vi "Martins HOT interface subtract and threshold.vi"() -> ()   [LabVIEW 2012] (continued)
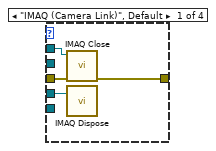
[diagram p2: hidden frame]
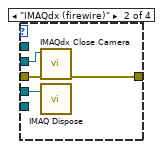
[diagram p3: hidden frame]
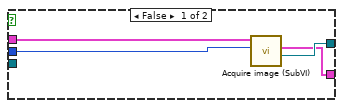
[diagram p6: hidden frame]
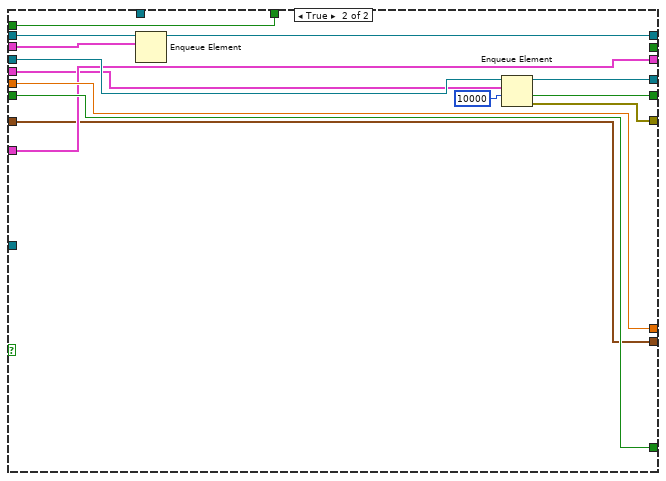
[diagram p18: hidden frame]
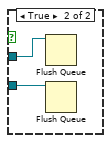
[diagram p19: hidden frame]
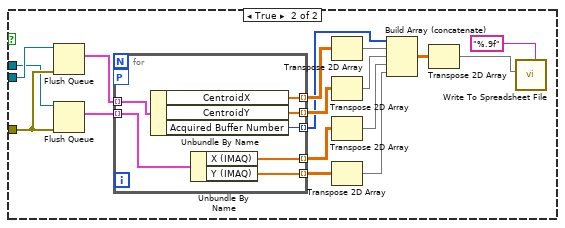
[diagram p20: hidden frame]
                  frame True {
                    n131 = local read "Coordinate mapping \n(IMAQ to SLM)"() -> (w402:T3)
                    n132 = call "Edit trap cluster.vi"("Coordinate mapping \n(IMAQ to SLM)"=w402, "trap cluster in"=w411) -> ("SubVI closed"=w406:bool, "Trap cluster out"=w405:T5)
                    n133 = Not(x=w406) -> (.not. x?=w401:bool)
                    n134 = call "Trap cluster 2 ROI.vi"("Trap cluster"=w405, "ROI in"=w403) -> ("ROI out"=w404:T2)  [unwired: 1 in]
                    n135 = property on="Monitor image" class="ImageControl"("ROI"=w404) -> ()  [unwired: 2 in, 2 out]
                    n136 = local write "Edit trap cluster"(w401) -> ()
                    n137 = Unbundle By Name(w405) -> ("Z"=w410:sgl[], "I"=w409:sgl[], "Group"=w407:bool[])
                  }
                }
                n138 = Unbundle By Name(w382) -> ("Trap number"=w381:i32[])
                n139 = case "Update display if\nnumber of traps \nhas changed" shown="True" w380 {
                  tunnel: w385 -> [_ w415]
                  tunnel: w383 -> [_ w414]
                  tunnel: w381 -> [_ w413]
                  tunnel: w378 -> [_ w412]
                  frame False {
                  }
                  frame True {
                    n140 = property on="I" class="Arr (strict)"("Value"=w414) -> ()  [unwired: 2 in, 2 out]
                    n141 = property on="Z" class="Arr (strict)"("Value"=w415) -> ()  [unwired: 2 in, 2 out]
                    n142 = property on="G" class="Arr (strict)"("Value"=w412) -> ()  [unwired: 2 in, 2 out]
                    "#" <- w413
                  }
                }
              }
              frame True {
                n143 = call "Move group.vi"("New handle position in"=w422, "Trap cluster in"=w424, "Previous handle position in"=w423, "Amplitudes"=w417, "Group"=w416, "Switch X/Y"=w418, "Move handle"=w419, "Z"=w420) -> ("Trap cluster out"=w421:T5)
              }
            }
            n144 = case shown="True" w359 {
              tunnel: w364 -> [_ w376]
              tunnel: w362 -> [w373 w375]
              tunnel: [w373 w374] -> w361
              frame False {
              }
              frame True {
                n145 = property on="Monitor image" class="ImageControl"(error in=w375, "ROI"=w376) -> (error out=w374:errorcluster)  [unwired: 1 in, 1 out]
              }
            }
          }
        }
        n146 = Wait (ms)(milliseconds to wait=u32 50) -> ()  [unwired: 1 out]
        n147 = Unbundle By Name("Path controls") -> ("Add current \npositions to path"=w341:bool, "Synchronize traps"=w350:bool, "Step length"=w353:dbl, "follow path"=w344:bool, "Arrive \nsimultaneously"=w352:bool)
        n148 = Or(x=w341, y=w350) -> (x .or. y?=w351:bool)
        n149 = Or(x=w350, y=w344) -> (x .or. y?=w348:bool)
        n150 = Or(x=w351, y=w344) -> (x .or. y?=w349:bool)
        n151 = case shown="True" "Create path" {
          tunnel: w356 -> [_ w437]
          tunnel: w346 -> [w425 w431]
          tunnel: w353 -> [_ w446]
          tunnel: w343 -> [_ w441]
          tunnel: w352 -> [_ w445]
          tunnel: w349 -> [_ w444]
          tunnel: w348 -> [_ w443]
          tunnel: w344 -> [_ w442]
          tunnel: w345 -> [w428 w438]
          tunnel: w340 -> [_ w436]
          tunnel: w339 -> [_ w435]
          tunnel: w337 -> [w427 w434]
          tunnel: [w427 w433] -> w336
          tunnel: "Updating trap cluster" -> [w426 _]
          tunnel: [w425 w432] -> w334
          frame False {
            n152 = case shown="True" w426 {
              tunnel: w425 -> [_ w430]
              tunnel: w428 -> [_ w429]
              frame False {
              }
              frame True {
                n153 = Lossy Enqueue Element(queue=w429, element=w430) -> ()  [unwired: 1 in, 4 out]
              }
            }
          }
          frame True {
            n154 = Lossy Enqueue Element "Enqueue\noverlay pos"(queue=w436, element=w431) -> ()  [unwired: 1 in, 4 out]
            n155 = case "Add wpt" shown="True" w444 {
              tunnel: w431 -> [_ w523]
              tunnel: w437 -> [w520 w524]
              tunnel: [w520 w521] -> w447
              tunnel: [_ w522] -> w439
              frame False {
              }
              frame True {
                n156 = Enqueue Element "Enqueue path\n waypts"(queue=w524, element=w523) -> (queue out=w521:refnum<queue>, error out=w522:errorcluster)  [unwired: 2 in, 1 out]
              }
            }
            n157 = case "Compute path" shown="True" w443 {
              tunnel: w447 -> [_ w531]
              tunnel: w441 -> [_ w530]
              tunnel: w446 -> [_ w529]
              tunnel: w445 -> [_ w528]
              tunnel: [w525 w526] -> w440
              tunnel: w439 -> [w525 w527]
              frame False {
              }
              frame True {
                n158 = call "compute path cluster.vi"("path queue"=w530, "Arrive simultaeously"=w528, "error in (no error)"=w527, "Step length\n(IMAQ pixels)"=w529, "waypoint queue"=w531) -> ("error out"=w526:errorcluster)  [unwired: 2 in]
              }
            }
            n159 = case "Follow path" shown="True" w442 {
              tunnel: w441 -> [_ w476]
              tunnel: w440 -> [_ w477]
              tunnel: w438 -> [_ w479]
              tunnel: w437 -> [_ w478]
              tunnel: w435 -> [_ w475]
              tunnel: w434 -> [w449 w456]
              tunnel: [w449 w455] -> w433
              tunnel: [w448 w450] -> w432
              tunnel: w431 -> [w448 _]
              frame False {
              }
              frame True {
                w470 = TRUE ("Visible")
                n160 = local write "Display path"(FALSE ("Display path")) -> ()
                n161 = Flush Queue "Flush Waypts"(queue=w478, error in (no error)=w477) -> (error out=w469:errorcluster)  [unwired: 2 out]
                n162 = Get Queue Status(queue=w476, error in (no error)=w469) -> (queue out=w473:refnum<queue>, error out=w468:errorcluster, # elements in queue=w472:i32)  [unwired: 1 in, 5 out]
                n163 = property on="Pause" class="Bool (strict)"(error in=w468, "Visible"=w470) -> (error out=w467:errorcluster)  [unwired: 1 in, 1 out]
                n164 = property on="cancel path" class="Bool"(error in=w467, "Visible"=w470) -> (error out=w466:errorcluster)  [unwired: 1 in, 1 out]
                n165 = for {
                  N: w472 -> [_]
                  tunnel: w466 -> [w498]
                  tunnel: w479 -> [w500]
                  tunnel: w473 -> [w496]
                  tunnel: [w496] -> w471
                  tunnel: [FALSE ("Group traps")] -> w451
                  shift-right: [w487] -> w450
                  shift-left: _ -> [w489]
                  tunnel: [w486] -> w465
                  tunnel: [w483] -> w463 mode=indexing
                  tunnel: [w484] -> w459
                  tunnel: [TRUE ("Display path")] -> w457
                  i -> [w484]
                  stop <- w493 stop-if-true
                  n166 = Dequeue Element(queue=w496, timeout in ms (-1)=0, error in (no error)=w498) -> (element=w488:T5, timed out?=w492:bool, error out=w499:errorcluster)  [unwired: 1 out]
                  n167 = while {
                    tunnel: [w517] -> w490
                    tunnel: ["cancel path"] -> w485
                    stop <- w519 stop-if-true
                    n168 = local read "Stop program"() -> (w517:bool)
                    n169 = Wait (ms)(milliseconds to wait="Step time \n(ms)") -> ()  [unwired: 1 out]
                    n170 = Or(x=w517, y="cancel path") -> (x .or. y?=w515:bool)
                    n171 = Implies(1:w515, 2:"Pause") -> (0:w519:bool)
                  }
                  n172 = case shown="True" "Skip step if \ntimed out" {
                    tunnel: w500 -> [w506 w511]
                    tunnel: w499 -> [w505 w509]
                    tunnel: [FALSE ("overflow?") w507] -> w491
                    tunnel: w488 -> [w504 w510]
                    tunnel: [w503 w508] -> w486
                    tunnel: 500 ("timeout in ms (-1)") -> [w502 _]
                    frame False {
                      n173 = Enqueue Element "Enqueue trap pos"(queue=w506, element=w504, timeout in ms (-1)=w502, error in (no error)=w505) -> (error out=w503:errorcluster)  [unwired: 2 out]
                    }
                    frame True {
                      n174 = Lossy Enqueue Element(queue=w511, element=w510, error in (no error)=w509) -> (overflow?=w507:bool, error out=w508:errorcluster)  [unwired: 2 out]
                    }
                  }
                  "Step skipped" <- w491
                  n175 = case shown="False" w490 {
                    tunnel: w489 -> [_ w513]
                    tunnel: w488 -> [w512 _]
                    tunnel: [w512 w513] -> w487
                    frame False {
                    }
                    frame True {
                    }
                  }
                  n176 = Or(x=w485, y=w490) -> (x .or. y?=w495:bool)
                  n177 = Or(x=w495, y=w492) -> (x .or. y?=w493:bool)
                  n178 = Tick Count (ms)() -> (millisecond timer value=w483:u32)
                }
                n179 = local read "Transpose SLM"() -> (w453:bool)
                n180 = call "Trap cluster 2 ROI.vi"("Switch X/Y"=w453, "Trap cluster"=w450, "ROI in"=w475) -> ("ROI out"=w474:T2)
                n181 = local write "Step skipped"(w451) -> ()
                n182 = local write "Create path"(w451) -> ()
                n183 = local write "Display path"(w457) -> ()
                n184 = local write "Group \nTraps"(w451) -> ()
                n185 = property on="Pause" class="Bool (strict)"(error in=w465, "Visible"=w451, "Value"=w451) -> (error out=w464:errorcluster)  [unwired: 1 in, 1 out]
                n186 = property on="cancel path" class="Bool"(error in=w464, "Visible"=w451) -> ()  [unwired: 1 in, 2 out]
                n187 = property on="follow path" class="Bool (strict)"("Value"=w451) -> ()  [unwired: 2 in, 2 out]
                n188 = property on="Monitor image" class="ImageControl"(error in=w456, "ROI"=w474) -> (error out=w455:errorcluster)  [unwired: 1 in, 1 out]
                n189 = Array Max & Min(array=w463) -> (max value=w462:u32, min value=w461:u32)  [unwired: 2 out]
                n190 = Subtract(x=w462, y=w461) -> (x-y=w460:u32)
                n191 = Increment(x=w459) -> (x+1=w454:i32)
                n192 = Divide(x=w460, y=w454) -> (x/y=→"Average step time (ms)":dbl)
                n193 = Flush Queue "Flush Path"(queue=w471) -> ()  [unwired: 1 in, 3 out]
              }
            }
          }
        }
        n194 = First Call?() -> (First Call?: T/F=w331:bool)
        n195 = Or(x="Apply Corrections", y=w331) -> (x .or. y?=w332:bool)
        n196 = case shown="True" w332 {
          frame False {
          }
          frame True {
            n197 = call "Apply Corrections.vi"() -> ()  [unwired: 1 in]
          }
        }
      }
      frame True {
        n198 = property on="Cancel calibration" class="Bool"("Visible"=w534) -> ()  [unwired: 2 in, 2 out]
        n199 = flat-sequence {
          tunnel: [w559] -> w546
          tunnel: [w561] -> w545
          tunnel: w541 -> [w559]
          tunnel: [w551] -> w540
          tunnel: [w548] -> w539
          tunnel: w538 -> [w553]
          tunnel: [w552] -> w536
          tunnel: [w624] -> w544
          tunnel: w546 -> [w624]
          tunnel: w545 -> [w582]
          tunnel: [w620] -> w543
          tunnel: w542 -> [w623]
          tunnel: w540 -> [w622]
          tunnel: w539 -> [w619]
          tunnel: [w618] -> w537
          tunnel: w536 -> [w618]
          tunnel: [w580] -> w532
          tunnel: w544 -> [w689]
          tunnel: w537 -> [w687]
          tunnel: [w686] -> w535
          frame #0 {
            w562 = u32 8 items=["Zoom Tool"=8, "Selection Tool"=0, "Pan Tool"=9, "Point Tool"=1, "Line Tool"=2, "Rectangle Tool"=3, "Rotated Rectangle Tool"=12, "Polyline Tool"=10, "Polygon Tool"=5, "Freehand Tool"=11, "Closed Freehand Tool"=6, "Ellipse Tool"=4, "Annulus Tool"=7] ("Current ROI Tool")
            n200 = local read "Using monitoring camera\nfor measurements"() -> (w547:bool)
            n201 = local read "Coordinate mapping \n(IMAQ to SLM)"() -> (w548:T3)
            n202 = Bundle By Name(cluster=w548, "sX"=0.0, "sY"=0.0, "cX"=1.0 ("sX"), "cY"=1.0) -> (w551:T3)
            n203 = case shown="False" w547 {
              frame False {
                n204 = call <vilib>:"Application Directory.vi"() -> ("Application Directory"=w565:path)
                n205 = Build Path(base path=w565, name or relative path="Sub VIs\\Display Image.vi") -> (appended path=w568:path)
                n206 = Open VI Reference(vi path=w568) -> (vi reference=w567:refnum<vi>)  [unwired: 5 in, 1 out]
                n207 = property class="VI"(reference=w567, "Front Panel.Open"=TRUE ("Front Panel Window:Open")) -> ()  [unwired: 1 in, 2 out]
              }
              frame True {
              }
            }
            n208 = local write "Coordinate mapping \n(IMAQ to SLM)"(w551) -> ()
            n209 = property on="ok" class="Bool"("Visible"=TRUE ("ROI Tool Buttons Visibile:Zoom Tool Button Visible")) -> ()  [unwired: 2 in, 2 out]
            n210 = property on="Monitor image" class="ImageControl"("Current ROI Tool"=w562) -> ()  [unwired: 2 in, 2 out]
            n211 = call <vilib>:"Three Button Dialog.vi"("Center Button Text (\"No\")"="Manual" ("T button name (\"OK\")"), "Left Button Text (\"Yes\")"="Auto" ("F button name (\"Cancel\")"), "message"="Mark the center of the \ndisplayed spot using the \nzoom and the point tool, \nthen click the OK button. \n(Will be repeated three times)") -> ("Which Button?"=w561:T13)  [unwired: 8 in]
            n212 = property on="Monitor image" class="ImageControl"(error in=w553, "ROI"=T2 {"Global Rectangle"=[100, 100, 394, 354], "Contours"=[{"Contour Type"=0, "ROI Type"=1, "Points"=[100, 100]}]} ("ROI 2")) -> (error out=w552:errorcluster)  [unwired: 1 in, 1 out]
          }
          frame #1 {
            w576 = sgl 0.0 ("sX")
            w577 = sgl 1.0 ("cX")
            n213 = local read "Coordinate mapping \n(Monitor to Measurement)"() -> (w575:T3)
            n214 = for {
              tunnel: [w645] -> w613 mode=indexing
              tunnel: [w644] -> w612 mode=indexing
              tunnel: T5[] [{"X (IMAQ)"=[-85.0], "Y (IMAQ)"=[-85.0], "Z"=[0.0], "I"=[100.0], "Trap number"=[0], "ROI number"=[0], "Number of traps"=1, "Group"=[]}, {"X (IMAQ)"=[85.0], "Y (IMAQ)"=[-85.0], "Z"=[0.0], "I"=[100.0], "Trap number"=[0], "ROI number"=[0], "Number of traps"=1, "Group"=[]}, {"X (IMAQ)"=[-85.0], "Y (IMAQ)"=[85.0], "Z"=[0.0], "I"=[100.0], "Trap number"=[0], "ROI number"=[0], "Number of traps"=0, "Group"=[]}] -> [w643] mode=indexing
              tunnel: [w640] -> w600 mode=indexing
              tunnel: [w638] -> w599 mode=indexing
              tunnel: w623 -> [w642]
              tunnel: [w637] -> w588 mode=indexing
              tunnel: [w636] -> w587 mode=indexing
              tunnel: w582 -> [w635]
              tunnel: [w633] -> w581
              stop <- w634 stop-if-true
              n215 = Enqueue Element "Enqueue trap pos"(queue=w642, element=w643) -> ()  [unwired: 2 in, 3 out]
              n216 = case shown="\"Left Button\", Default" w635 {
                tunnel: [w650 w667 _ _] -> w645
                tunnel: [w649 w666 _ _] -> w644
                tunnel: [w646 w664 w677 w678] -> w634
                tunnel: [w648 w661 _ _] -> w637
                tunnel: [w647 w660 _ _] -> w636
                tunnel: [w646 w659 w677 w678] -> w633
                frame "Left Button", Default {
                  n217 = flat-sequence {
                    tunnel: [w658] -> w650
                    tunnel: [w657] -> w649
                    tunnel: [w656] -> w648
                    tunnel: [w655] -> w647
                    tunnel: [FALSE] -> w646
                    frame #0 {
                      n218 = Wait (ms)(milliseconds to wait=u32 300) -> ()  [unwired: 1 out]
                    }
                    frame #1 {
                      n219 = local read "Monitoring image"() -> (w654:T1)
                      n220 = local read "Measurement image"() -> (w653:T1)
                      n221 = call "Find spot in image.vi"("Image"=w654) -> ("Y Centroid"=w657:dbl, "X Centroid"=w658:dbl)  [unwired: 7 in]
                      n222 = call "Find spot in image.vi"("Image"=w653) -> ("Y Centroid"=w655:dbl, "X Centroid"=w656:dbl)  [unwired: 7 in]
                    }
                  }
                }
                frame "Center Button" {
                  n223 = while {
                    tunnel: [w675] -> w665
                    tunnel: [w672] -> w664
                    tunnel: [w670] -> w663
                    tunnel: [w669] -> w659
                    stop <- w673 stop-if-true
                    n224 = local read "Stop program"() -> (w669:bool)
                    n225 = global read "Global variables.vi" "Measurement ROI"() -> (w670:T14)
                    n226 = Wait (ms)(milliseconds to wait=u32 50) -> ()  [unwired: 1 out]
                    n227 = Or(x=w669, y="Cancel calibration") -> (x .or. y?=w672:bool)
                    n228 = property on="Monitor image" class="ImageControl"() -> ("ROI"=w675:T2)  [unwired: 2 in, 2 out]
                    n229 = Or(x="ok", y=w672) -> (x .or. y?=w673:bool)
                  }
                  n230 = Unbundle By Name(w663) -> ("Global Rectangle"=w662:i32[])  [unwired: 1 out]
                  n231 = Unbundle By Name(w665) -> ("Global Rectangle"=w668:i32[])  [unwired: 1 out]
                  n232 = Index Array(array=w668) -> (element #1=w667:i32, element #2=w666:i32)  [unwired: 2 in]
                  n233 = Index Array(array=w662) -> (element #1=w661:i32, element #2=w660:i32)  [unwired: 2 in]
                }
                frame "Right Button" {
                  w677 = TRUE
                }
                frame "Window Close" {
                  w678 = TRUE
                }
              }
              n234 = Unbundle By Name(w643) -> ("X (IMAQ)"=w641:sgl[], "Y (IMAQ)"=w639:sgl[])
              n235 = Index Array(array=w639) -> (element=w638:sgl)  [unwired: 1 in]
              n236 = Index Array(array=w641) -> (element=w640:sgl)  [unwired: 1 in]
            }
            n237 = Index Array(array=w612) -> (element #1=w614:dbl, element #2=w615:dbl)  [unwired: 2 in]
            n238 = Index Array(array=w613) -> (element #1=w616:dbl, element #2=w617:dbl)  [unwired: 2 in]
            n239 = Subtract(x=w617, y=w616) -> (x-y=w609:dbl)
            n240 = Subtract(x=w615, y=w614) -> (x-y=w607:dbl)
            n241 = Absolute Value(x=w607) -> (abs(x)=w606:dbl)
            n242 = Absolute Value(x=w609) -> (abs(x)=w608:dbl)
            n243 = Less?(x=w608, y=w606) -> (x < y?=w571:bool)
            n244 = case shown="False" w571 {
              tunnel: w613 -> [w630 w632]
              tunnel: w612 -> [w629 w631]
              tunnel: [w629 w632] -> w610
              tunnel: [w630 w631] -> w611
              frame False {
              }
              frame True {
              }
            }
            n245 = Index Array(array=w587) -> (element #1=w592:dbl, element #2=w591:dbl)  [unwired: 2 in]
            n246 = Index Array(array=w588) -> (element #1=w590:dbl, element #2=w589:dbl)  [unwired: 2 in]
            n247 = Subtract(x=w589, y=w590) -> (x-y=w593:dbl)
            n248 = Subtract(x=w591, y=w592) -> (x-y=w595:dbl)
            n249 = Absolute Value(x=w595) -> (abs(x)=w596:dbl)
            n250 = Absolute Value(x=w593) -> (abs(x)=w594:dbl)
            n251 = Less?(x=w594, y=w596) -> (x < y?=w572:bool)
            n252 = case shown="True" w572 {
              tunnel: w588 -> [w626 w628]
              tunnel: w587 -> [w625 w627]
              tunnel: [w625 w628] -> w597
              tunnel: [w626 w627] -> w598
              frame False {
              }
              frame True {
              }
            }
            n253 = formula code="cX = (xSLM[1] - xSLM[0]) / (xMonitor[1] - xMonitor[0]); \ncY = (ySLM[2] - ySLM[0]) / (yMonitor[2] - yMonitor[0]); \n\nsX = xSLM[0] - xMonitor[0] *cX;\nsY = ySLM[0] - yMonitor[0] *cY;\n\ncXm = (xMeasure[1] - xMeasure[0]) / (xMonitor[1] - xMonitor[0]); \ncYm = (yMeasure[2] - yMeasure[0]) / (yMonitor[2] - yMonitor[0]); \n\nsXm = xMeasure[0] - xMonitor[0] *cXm;\nsYm = yMeasure[0] - yMonitor[0] *cYm;"("xMonitor"=w611, "yMonitor"=w610, "xSLM"=w600, "ySLM"=w599, "xMeasure"=w598, "yMeasure"=w597) -> ("cX"=w605:dbl, "cY"=w604:dbl, "sX"=w603:dbl, "sY"=w602:dbl, "cXm"=w586:dbl, "cYm"=w585:dbl, "sXm"=w584:dbl, "sYm"=w583:dbl)
            n254 = local read "Using monitoring camera\nfor measurements"() -> (w570:bool)
            n255 = Select(t=FALSE, s=w570, f=w572) -> (s? t:f=w573:bool)
            n256 = Bundle By Name(cluster=w622, "cX"=w605, "cY"=w604, "sX"=w603, "sY"=w602) -> (w621:T3)
            n257 = Bundle By Name(cluster=w575, "cX"=w577, "cY"=w577, "sX"=w576, "sY"=w576) -> (w574:T3)
            n258 = Bundle By Name(cluster=w575, "cX"=w586, "cY"=w585, "sX"=w584, "sY"=w583) -> (w578:T3)
            n259 = Select(t=w574, s=w570, f=w578) -> (s? t:f=w579:T3)
            n260 = case "Calibration canceled?" shown="False" w581 {
              tunnel: w621 -> [w682 _]
              tunnel: [w682 w684] -> w620
              tunnel: w619 -> [_ w684]
              tunnel: [w679 w683] -> w580
              tunnel: w579 -> [w679 w683]
              tunnel: w573 -> [w681 _]
              tunnel: w571 -> [w680 _]
              frame False {
                n261 = local write "Transpose Measurement"(w681) -> ()
                n262 = local write "Transpose SLM"(w680) -> ()
              }
              frame True {
              }
            }
          }
          frame #2 {
            w685 = FALSE ("ROI Tool Buttons Visibile:Zoom Tool Button Visible")
            w688 = u32 1 items=["Zoom Tool"=8, "Selection Tool"=0, "Pan Tool"=9, "Point Tool"=1, "Line Tool"=2, "Rectangle Tool"=3, "Rotated Rectangle Tool"=12, "Polyline Tool"=10, "Polygon Tool"=5, "Freehand Tool"=11, "Closed Freehand Tool"=6, "Ellipse Tool"=4, "Annulus Tool"=7] ("Current ROI Tool")
            n263 = property on="Monitor image" class="ImageControl"(error in=w687, "ROI"=w689) -> (error out=w686:errorcluster)  [unwired: 1 in, 1 out]
            n264 = property on="Monitor image" class="ImageControl"("Current ROI Tool"=w688, "Point Tool Button Visibile"=w685) -> ()  [unwired: 2 in, 2 out]
            n265 = property on="Cancel" class="Bool"("Visible"=w685) -> ()  [unwired: 2 in, 2 out]
            n266 = property on="ok" class="Bool"("Visible"=w685) -> ()  [unwired: 2 in, 2 out]
          }
        }
        n267 = local write "Coordinate mapping \n(IMAQ to SLM)"(w543) -> ()
        n268 = local write "Coordinate mapping \n(Monitor to Measurement)"(w532) -> ()
      }
    }
  }
  n269 = while "User input and events loop" {
    tunnel: w73 -> [w708]
    tunnel: w12 -> [w697]
    tunnel: w47 -> [w696]
    tunnel: w11 -> [w695]
    tunnel: [w694] -> w56
    tunnel: w55 -> [w693]
    tunnel: [w692] -> w54
    tunnel: w37 -> [w690]
    stop <- w700 stop-if-true
    w705 = u32 8 items=["Zoom Tool"=8, "Selection Tool"=0, "Pan Tool"=9, "Point Tool"=1, "Line Tool"=2, "Rectangle Tool"=3, "Rotated Rectangle Tool"=12, "Polyline Tool"=10, "Polygon Tool"=5, "Freehand Tool"=11, "Closed Freehand Tool"=6, "Ellipse Tool"=4, "Annulus Tool"=7] ("Current ROI Tool")
    w702 = T15 [enum."LCONTROL"] items=["0", "1", "2", "3", "4", "5", "6", "7", "8", "9", "A", "B", "C", "D", "E", "F", "G", "H", "I", "J", "K", "L", "M", "N", "O", "P", "Q", "R", "S", "T", "U", "V", "W", "X", "Y", "Z", "F1", "F2", "F3", "F4", "F5", "F6", "F7", "F8", "F9", "F10", "F11", "F12", "F13", "F14", "F15", "ADD", "BACK", "BACKSLASH", "CAPITAL", "COMMA", "DECIMAL", "DELETE", "DIVIDE", "DOWN", "END", "EQUALS", "ESCAPE", "GRAVE (`)", "HOME", "INSERT", "LBRACKET", "LCONTROL", "LEFT", "L ALT", "LSHIFT", "LWIN", "MINUS", "MULTIPLY", "NEXT", "NUMLOCK", "NUMPAD_0", "NUMPAD_1", "NUMPAD_2", "NUMPAD_3", "NUMPAD_4", "NUMPAD_5", "NUMPAD_6", "NUMPAD_7", "NUMPAD_8", "NUMPAD_9", "PAUSE", "PERIOD", "PRIOR (PG UP)", "RBRACKET", "RCONTROL", "RETURN", "RIGHT", "R ALT", "RSHIFT", "RWIN", "SCROLL", "SEMICOLON", "SLASH", "SPACE", "SUBTRACT", "TAB", "UP", "ENTER (num pad)", "' (quote)"] ("keys pressed")
    n270 = call-poly <vilib>:"Acquire Input Data.vi"("device ID"=w708, "error in (no error)"=w693) -> ("device ID"=w694:refnum<k1>, "keys pressed"=w701:T15, "error out"=w692:errorcluster)  [unwired: 15 out]
    n271 = property on="Monitor image" class="ImageControl"() -> ("Current ROI Tool"=w704:u32)  [unwired: 2 in, 2 out]
    n272 = Equal?(x=w701, y=w702) -> (x = y?=w703:bool[])
    n273 = Not Equal?(x=w704, y=w705) -> (x != y?=w706:bool)
    n274 = Or Array Elements(Boolean array=w703) -> (logical OR=w707:bool)
    n275 = case shown="True" w706 {
      tunnel: w707 -> [_ w753]
      frame False {
      }
      frame True {
        n276 = case shown="False" w753 {
          frame False {
            w754 = u32 0 items=["Zoom Tool"=8, "Selection Tool"=0, "Pan Tool"=9, "Point Tool"=1, "Line Tool"=2, "Rectangle Tool"=3, "Rotated Rectangle Tool"=12, "Polyline Tool"=10, "Polygon Tool"=5, "Freehand Tool"=11, "Closed Freehand Tool"=6, "Ellipse Tool"=4, "Annulus Tool"=7] ("Current ROI Tool")
            n277 = property on="Monitor image" class="ImageControl"("Current ROI Tool"=w754) -> ()  [unwired: 2 in, 2 out]
          }
          frame True {
            w755 = u32 1 items=["Zoom Tool"=8, "Selection Tool"=0, "Pan Tool"=9, "Point Tool"=1, "Line Tool"=2, "Rectangle Tool"=3, "Rotated Rectangle Tool"=12, "Polyline Tool"=10, "Polygon Tool"=5, "Freehand Tool"=11, "Closed Freehand Tool"=6, "Ellipse Tool"=4, "Annulus Tool"=7] ("Current ROI Tool")
            n278 = property on="Monitor image" class="ImageControl"("Current ROI Tool"=w755) -> ()  [unwired: 2 in, 2 out]
          }
        }
      }
    }
    n279 = Wait (ms)(milliseconds to wait=u32 50) -> ()  [unwired: 1 out]
    n280 = case shown="False" "View Licence" {
      frame False {
      }
      frame True {
        n281 = call "View license.vi"() -> ()  [unwired: 1 in]
      }
    }
    n282 = event shown="[0] Timeout" {
      selector: _ -> [_ _ _ _ _ _ _ _ _ _ _]
      dyn-events: _ -> [_ _ _ _ _ _ _ _ _ _ _]
      timeout: 0 -> [_ _ _ _ _ _ _ _ _ _ _]
      tunnel: w697 -> [_ _ w719 _ _ _ _ _ _ _ _]
      tunnel: w696 -> [_ _ w718 _ _ _ _ _ _ _ _]
      tunnel: w695 -> [_ _ w722 _ _ _ _ _ _ _ _]
      tunnel: w690 -> [_ _ _ _ _ _ w735 _ _ _ _]
      event Timeout {
        n283 = event-data() -> ()  [unwired: 1 in, 2 out]
      }
      event "Display hologram\nand computed \nimage plane": Value Change {
        n284 = event-data() -> ("NewVal"=w710:bool)  [unwired: 1 in, 4 out]
        n285 = property on="Current trap pos" class="Clust (strict)"("Visible"=w710) -> ()  [unwired: 2 in, 2 out]
        n286 = property on="Displayed Hologram" class="IntGraph (strict)"("Visible"=w710) -> ()  [unwired: 2 in, 2 out]
        n287 = property on="Calculated image plane" class="IntGraph (strict)"("Visible"=w710) -> ()  [unwired: 2 in, 2 out]
        n288 = property on="Property Node" class="VI"() -> ("Front Panel.WinBounds"=w717:T16)  [unwired: 2 in, 2 out]
        n289 = Unbundle By Name(w717) -> ("Right"=w716:i16, "Left"=w715:i16)
        n290 = Subtract(x=w716, y=w715) -> (x-y=w714:i16)
        n291 = Select(t=i16 500 ("x-y"), s=w710, f=i16 196 ("x-y")) -> (s? t:f=w709:i16)
        n292 = Subtract(x=w714, y=w709) -> (x-y=w713:i16)
        n293 = property on="Splitter" class="Splitter"("Position"=w713) -> ()  [unwired: 2 in, 2 out]
      }
      event "Create path": Value Change {
        n294 = event-data() -> ()  [unwired: 1 in, 5 out]
        n295 = property on="follow path" class="Bool (strict)"("Value"=FALSE) -> ()  [unwired: 2 in, 2 out]
        n296 = Flush Queue "Flush path \nwaypt queue"(queue=w718) -> ()  [unwired: 1 in, 3 out]
        n297 = Preview Queue Element(queue=w719) -> (element=w720:T5, error out=w723:errorcluster)  [unwired: 2 in, 2 out]
        n298 = Flush Queue "Flush path queue"(queue=w722) -> (queue out=w721:refnum<queue>)  [unwired: 1 in, 2 out]
        n299 = Enqueue Element "Enqueue current \ntrap pos in path"(queue=w721, element=w720) -> ()  [unwired: 2 in, 3 out]
        n300 = Enqueue Element "Enqueue current \ntrap pos in path \nwaypts"(queue=w718, element=w720, error in (no error)=w723) -> ()  [unwired: 1 in, 3 out]
      }
      event "cancel path": Value Change {
        n301 = event-data() -> ()  [unwired: 1 in, 5 out]
        n302 = local write "Create path"(FALSE ("Visible")) -> ()
      }
      event "Monitor image", "Group \nTraps", "Z", "I", "Coordinate mapping \n(IMAQ to SLM)": Mouse Down {
        w726 = FALSE ("Edit trap cluster")
        n303 = event-data() -> ()  [unwired: 1 in, 7 out]
        n304 = local write "Updating trap cluster"(TRUE ("Update trap positions")) -> ()
        n305 = local write "Edit trap cluster"(w726) -> ()
        n306 = call <vilib>:"Application Directory.vi"() -> ("Application Directory"=w727:path)
        n307 = Build Path(base path=w727, name or relative path="Sub VIs\\Edit trap cluster.vi") -> (appended path=w730:path)
        n308 = Open VI Reference(vi path=w730) -> (vi reference=w729:refnum<vi>)  [unwired: 5 in, 1 out]
        n309 = property class="VI"(reference=w729, "Front Panel.Open"=w726) -> ()  [unwired: 1 in, 2 out]
      }
      event "Group \nTraps", "Z", "I", "Monitor image", "Coordinate mapping \n(IMAQ to SLM)": Mouse Up {
        n310 = event-data() -> ()  [unwired: 1 in, 7 out]
        n311 = flat-sequence {
          frame #0 {
            n312 = Wait (ms)(milliseconds to wait=u32 100) -> ()  [unwired: 1 out]
          }
          frame #1 {
            n313 = local write "Updating trap cluster"(FALSE ("Update trap positions")) -> ()
          }
        }
      }
      event "Record": Value Change {
        n314 = event-data() -> ()  [unwired: 1 in, 5 out]
        n315 = Unbundle By Name(w735) -> ("Image buffers"=w734:T1[])
        n316 = for {
          tunnel: w734 -> [w736] mode=indexing
          n317 = call "IMAQ Clear Overlay"("Image"=w736) -> ()  [unwired: 9 in, 2 out]
        }
      }
      event "Display data": Value Change {
        n318 = event-data() -> ("NewVal"=w738:bool)  [unwired: 1 in, 4 out]
        n319 = call <vilib>:"Application Directory.vi"() -> ("Application Directory"=w737:path)
        n320 = Build Path(base path=w737, name or relative path="Sub VIs\\Display Cetroids (SubVI).vi") -> (appended path=w741:path)
        n321 = Open VI Reference(vi path=w741) -> (vi reference=w740:refnum<vi>)  [unwired: 5 in, 1 out]
        n322 = property class="VI"(reference=w740, "Front Panel.Open"=w738) -> ()  [unwired: 1 in, 2 out]
      }
      event "Display ROIs": Value Change {
        n323 = event-data() -> ("NewVal"=w742:bool)  [unwired: 1 in, 4 out]
        n324 = call <vilib>:"Application Directory.vi"() -> ("Application Directory"=w743:path)
        n325 = Build Path(base path=w743, name or relative path="Sub VIs\\Display ROIs.vi") -> (appended path=w746:path)
        n326 = Open VI Reference(vi path=w746) -> (vi reference=w745:refnum<vi>)  [unwired: 5 in, 1 out]
        n327 = property class="VI"(reference=w745, "Front Panel.Open"=w742) -> ()  [unwired: 1 in, 2 out]
      }
      event "Display ROIs": Value Change {
        n328 = event-data() -> ("NewVal"=w747:bool)  [unwired: 1 in, 4 out]
        n329 = call <vilib>:"Application Directory.vi"() -> ("Application Directory"=w748:path)
        n330 = Build Path(base path=w748, name or relative path="Sub VIs\\Display Image.vi") -> (appended path=w751:path)
        n331 = Open VI Reference(vi path=w751) -> (vi reference=w750:refnum<vi>)  [unwired: 5 in, 1 out]
        n332 = property class="VI"(reference=w750, "Front Panel.Open"=w747) -> ()  [unwired: 1 in, 2 out]
      }
      event "Edit trap cluster": Value Change {
        n333 = event-data() -> ("NewVal"=w752:bool)  [unwired: 1 in, 4 out]
        n334 = local write "Updating trap cluster"(w752) -> ()
      }
    }
    n335 = local read "Stop program"() -> (w700:bool)
  }
  n336 = Unbundle By Name(w26) -> ("Camera type"=w16:T8)
  n337 = local read "Using monitoring camera\nfor measurements"() -> (w15:bool)
  n338 = call "IMAQ Create"("Image Name"="Monitoring copy", "Image Type"=w6) -> ("New Image"=w13:T1)  [unwired: 3 in, 1 out]
  n339 = while {
    tunnel: w26 -> [w773]
    tunnel: [w771] -> w17
    tunnel: w16 -> [w772]
    tunnel: w15 -> [w769]
    tunnel: w13 -> [w768]
    tunnel: w12 -> [w767]
    tunnel: w11 -> [w761]
    tunnel: w10 -> [w756]
    stop <- w774 stop-if-true
    n340 = Preview Queue Element(queue=w767, timeout in ms (-1)=10) -> (element=w766:T5)  [unwired: 1 in, 3 out]
    n341 = case shown="True" w769 {
      tunnel: w773 -> [w779 w782]
      tunnel: w772 -> [w778 _]
      tunnel: [w777 w783] -> w765
      tunnel: [w776 w780] -> w771
      tunnel: w768 -> [_ w785]
      frame False {
        n342 = call "Acquire image (SubVI).vi"("Camera type"=w778, "Measurement camera \ncluster in"=w779) -> ("Image Out"=w777:T1, "Measurement camera cluster out"=w776:T10)  [unwired: 7 in, 1 out]
      }
      frame True {
        n343 = Unbundle By Name(w782) -> ("Image"=w786:T1, "Camera error"=w784:errorcluster)
        n344 = call "IMAQ Copy"("error in (no error)"=w784, "Image Dst"=w785, "Image Src"=w786) -> ("error out"=w781:errorcluster, "Image Dst Out"=w783:T1)  [unwired: 3 in]
        n345 = Bundle By Name(cluster=w782, "Camera error"=w781) -> (w780:T10)
      }
    }
    n346 = Wait (ms)(milliseconds to wait=u32 200) -> ()  [unwired: 1 out]
    n347 = local read "Stop program"() -> (w774:bool)
    n348 = local read "ROI size"() -> (w764:dbl)
    n349 = Get Queue Status(queue=w761, return elements? (F)="Display path") -> (elements=w762:T5[])  [unwired: 1 in, 7 out]
    n350 = local read "Transpose SLM"() -> (w763:bool)
    n351 = case shown="True" "Display ROIs" {
      tunnel: w756 -> [_ w775]
      frame False {
      }
      frame True {
        n352 = call "Display ROIs.vi"("ROI array in"=w775) -> ()  [unwired: 11 in]
      }
    }
    n353 = call "Create trap overlay.vi"("Current trap cluster"=w766, "Image in"=w765, "ROI size"=w764, "Switch X/Y"=w763, "Path"=w762) -> ("Image Out"=→"Monitor image":T1)
  }
  n354 = Unbundle By Name(w17) -> ("Camera type"=w23:T8, "IMAQ Session"=w22:refnum<k11>, "IMAQdx Session"=w21:T9, "Camera error"=w20:errorcluster, "Image"=w19:T1, "Image buffers"=w18:T1[])
  n355 = case shown="\"IMAQ ring\"" w23 {
    tunnel: w22 -> [w790 _ _ w799]
    tunnel: [w789 w794 w795 w798] -> _
    tunnel: w21 -> [_ w793 _ _]
    tunnel: w20 -> [w788 w792 w795 w797]
    tunnel: w19 -> [w787 w791 _ _]
    tunnel: w18 -> [_ _ _ w796]
    frame "IMAQ (Camera Link)", Default {
      n356 = call <vilib>:"IMAQ Close.vi"("error in (no error)"=w788, "IMAQ Session In"=w790) -> ("error out"=w789:errorcluster)  [unwired: 9 in]
      n357 = call "IMAQ Dispose"("Image"=w787) -> ()  [unwired: 5 in, 1 out]
    }
    frame "IMAQdx (firewire)" {
      n358 = call <vilib>:"IMAQdx Close Camera.vi"("error in"=w792, "Session In"=w793) -> ("error out"=w794:errorcluster)  [unwired: 9 in]
      n359 = call "IMAQ Dispose"("Image"=w791) -> ()  [unwired: 5 in, 1 out]
    }
    frame "No camera" {
    }
    frame "IMAQ ring" {
      n360 = call <vilib>:"IMAQ Close.vi"("error in (no error)"=w797, "IMAQ Session In"=w799) -> ("error out"=w798:errorcluster)  [unwired: 9 in]
      n361 = for {
        tunnel: w796 -> [w800] mode=indexing
        n362 = call "IMAQ Dispose"("Image"=w800) -> ()  [unwired: 5 in, 1 out]
      }
    }
  }
  n363 = call "FreeGPUandSLM.vi"("error in"=w35) -> ("error out"=w58:errorcluster)  [unwired: 1 out]
  "CUDA/SLM error" <- w58
  n364 = call-poly <vilib>:"Close Input Device.vi"("error in (no error)"=w54, "device ID"=w56) -> ()  [unwired: 9 out]
  n365 = Unbundle By Name(w29) -> ("Camera type"=w33:T8, "IMAQ Session"=w32:refnum<k11>, "IMAQdx Session"=w31:T9, "Camera error"=w30:errorcluster, "Image"=w28:T1, "Image buffers"=w27:T1[])
  n366 = case shown="\"IMAQ ring\"" w33 {
    tunnel: w32 -> [w804 _ _ w813]
    tunnel: [w803 w808 w809 w812] -> w60
    tunnel: w31 -> [_ w807 _ _]
    tunnel: w30 -> [w802 w806 w809 w811]
    tunnel: w28 -> [w801 w805 _ _]
    tunnel: w27 -> [_ _ _ w810]
    frame "IMAQ (Camera Link)", Default {
      n367 = call <vilib>:"IMAQ Close.vi"("error in (no error)"=w802, "IMAQ Session In"=w804) -> ("error out"=w803:errorcluster)  [unwired: 9 in]
      n368 = call "IMAQ Dispose"("Image"=w801) -> ()  [unwired: 5 in, 1 out]
    }
    frame "IMAQdx (firewire)" {
      n369 = call <vilib>:"IMAQdx Close Camera.vi"("error in"=w806, "Session In"=w807) -> ("error out"=w808:errorcluster)  [unwired: 9 in]
      n370 = call "IMAQ Dispose"("Image"=w805) -> ()  [unwired: 5 in, 1 out]
    }
    frame "No camera" {
    }
    frame "IMAQ ring" {
      n371 = for {
        tunnel: w810 -> [w814] mode=indexing
        n372 = call "IMAQ Dispose"("Image"=w814) -> ()  [unwired: 5 in, 1 out]
      }
      n373 = call <vilib>:"IMAQ Close.vi"("error in (no error)"=w811, "IMAQ Session In"=w813) -> ("error out"=w812:errorcluster)  [unwired: 9 in]
    }
  }
  n374 = Unbundle By Name(w61) -> ("Contours"=w66:T17)
  n375 = Index Array(array=w66) -> (element=w65:T18)  [unwired: 1 in]
  n376 = Merge Errors(w60, w59) -> (w57:errorcluster)
  "NI Vision error" <- w57
  n377 = flat-sequence {
    tunnel: w58 -> [_]
    tunnel: w57 -> [_]
    frame #0 {
      n378 = local write "Stop program"(FALSE ("Stop program")) -> ()
    }
  }
  n379 = Unbundle By Name(w65) -> ("ROI Type"=w64:u32)
  n380 = Equal?(x=w64, y=u32 1) -> (x = y?=w62:bool)
  n381 = case shown="True" w62 {
    tunnel: w61 -> [_ w816]
    frame False {
    }
    frame True {
      n382 = local write "ROI"(w816) -> ()
    }
  }
